vi "UHR-Fleezers Control (host) - 12.0(oscillate_test).vi"() -> ()   [LabVIEW 2014] (continued)
        n1707 = Concatenate Strings("User: ", "User", "\r", "Parameters saved.") -> (w2416:string)
        n1708 = call "Update messages.vi"("Message to add"=w2416, "Old message string"=w2421) -> ("New message string"=w2415:string)
        n1709 = local write "Messages"(w2415) -> ()
      }
      event "Load user params": Value Change {
        n1710 = event-data() -> ()  [unwired: 7 out]
        n1711 = local write "Load user params"(FALSE ("Read user\nparams")) -> ()
        n1712 = flat-sequence {
          tunnel: [w2453] -> w2441
          tunnel: [w2452] -> w2439
          tunnel: [w2451] -> w2437
          tunnel: [w2450] -> w2435
          tunnel: [w2449] -> w2433
          tunnel: [w2448] -> w2431
          tunnel: [w2447] -> w2429
          tunnel: [w2446] -> w2427
          tunnel: [w2445] -> w2425
          tunnel: [w2444] -> w2423
          tunnel: [w2463] -> w2442
          tunnel: w2441 -> [w2463]
          tunnel: [w2462] -> w2440
          tunnel: w2439 -> [w2462]
          tunnel: [w2461] -> w2438
          tunnel: w2437 -> [w2461]
          tunnel: [w2460] -> w2436
          tunnel: w2435 -> [w2460]
          tunnel: [w2459] -> w2434
          tunnel: w2433 -> [w2459]
          tunnel: [w2458] -> w2432
          tunnel: w2431 -> [w2458]
          tunnel: [w2457] -> w2430
          tunnel: w2429 -> [w2457]
          tunnel: [w2456] -> w2428
          tunnel: w2427 -> [w2456]
          tunnel: [w2455] -> w2426
          tunnel: w2425 -> [w2455]
          tunnel: [w2454] -> w2424
          tunnel: w2423 -> [w2454]
          tunnel: w2442 -> [w2480]
          tunnel: w2440 -> [w2479]
          tunnel: w2438 -> [w2478]
          tunnel: w2436 -> [w2477]
          tunnel: w2434 -> [w2476]
          tunnel: w2432 -> [w2475]
          tunnel: w2430 -> [w2474]
          tunnel: w2428 -> [w2473]
          tunnel: w2426 -> [w2472]
          tunnel: w2424 -> [w2471]
          frame #0 {
            # "Make exceptions.\nThese will not be\nloaded."
            n1713 = local read "Sample Channel\nFlow"() -> (w2448:bool)
            n1714 = local read "Green ON/Interlacing"() -> (w2449:bool)
            n1715 = local read "Trap 1 (ON/OFF)"() -> (w2453:bool)
            n1716 = local read "Trap 2 (ON/OFF)"() -> (w2452:bool)
            n1717 = local read "Trap Pos. FB ON"() -> (w2444:bool)
            n1718 = local read "Inject Pump 1"() -> (w2447:bool)
            n1719 = local read "Inject Pump 3"() -> (w2446:bool)
            n1720 = local read "Trap D (MHz)"() -> (w2445:dbl)
            n1721 = local read "Index"() -> (w2450:dbl)
            n1722 = local read "Fish"() -> (w2451:bool)
          }
          frame #1 {
            n1723 = local read "User"() -> (w2464:string)
            n1724 = call "retrieve control values.vi"("User"=w2464) -> ()  [unwired: 10 in, 1 out]
            n1725 = local read "Messages"() -> (w2470:string)
            n1726 = Concatenate Strings("User: ", w2464, "\r", "Parameters loaded.") -> (w2465:string)
            n1727 = call "Update messages.vi"("Message to add"=w2465, "Old message string"=w2470) -> ("New message string"=w2469:string)
            n1728 = local write "Messages"(w2469) -> ()
          }
          frame #2 {
            n1729 = local write "Sample Channel\nFlow"(w2475) -> ()
            n1730 = local write "Green ON/Interlacing"(w2476) -> ()
            n1731 = local write "Trap 1 (ON/OFF)"(w2480) -> ()
            n1732 = local write "Trap 2 (ON/OFF)"(w2479) -> ()
            n1733 = local write "Inject Pump 1"(w2474) -> ()
            n1734 = local write "Trap Pos. FB ON"(w2471) -> ()
            n1735 = local write "Inject Pump 3"(w2473) -> ()
            n1736 = local write "Trap D (MHz)"(w2472) -> ()
            n1737 = local write "Index"(w2477) -> ()
            n1738 = local write "Fish"(w2478) -> ()
          }
        }
      }
      event "Abort wiggle": Value Change {
        n1739 = event-data() -> ()  [unwired: 7 out]
        n1740 = flat-sequence {
          tunnel: w2484 -> [w2488]
          tunnel: w2483 -> [w2487]
          tunnel: [w2486] -> w2481
          tunnel: [w2490] -> w2482
          tunnel: w2481 -> [w2490]
          frame #0 {
            n1741 = xnode "Read/Write Control"("FPGA VI Reference In"=w2488, "error in"=w2487, "Abort wiggle 1"="Abort wiggle", "Abort wiggle 2"="Abort wiggle") -> ("error out"=w2486:errorcluster)  [unwired: 1 out]
          }
          frame #1 {
            n1742 = local write "Abort wiggle"(FALSE ("Abort wiggle")) -> ()
          }
        }
      }
    }
    "error out 2" <- w1261
    n1743 = node-c288() -> ()  [unwired: 2 out]
  }
  n1744 = node-c288() -> (w126:T26)  [unwired: 4 in]
  n1745 = local write "Target size"(cluster{"Width":dbl, "Height":dbl} {"Width"=40.0, "Height"=40.0} ("Target size")) -> ()
  n1746 = timed-loop "Run Scripts, including: stage motion" {
    tunnel: w130 -> [w2498]
    tunnel: w5 -> [w2499]
    tunnel: [w2499] -> w129
    tunnel: [w2498] -> w128
    timing: w126 -> [_]
    timing-out: [_] -> w125
    tunnel: w111 -> [w2497]
    tunnel: w112 -> [w2496]
    tunnel: w55 -> [w2493]
    tunnel: w54 -> [w2492]
    tunnel: w53 -> [w2494]
    tunnel: w52 -> [w2495]
    stop <- w2491 stop-if-true
    n1747 = node-c288() -> ()  [unwired: 1 in, 1 out]
    n1748 = event shown="[12] \"Got ADig bead\": Value Change" {
      selector: _ -> [_ _ _ _ _ _ _ _ _ _ _ _ _ _ _ _ _ _ _ _ _]
      dyn-events: _ -> [_ _ _ _ _ _ _ _ _ _ _ _ _ _ _ _ _ _ _ _ _]
      timeout: _ -> [_ _ _ _ _ _ _ _ _ _ _ _ _ _ _ _ _ _ _ _ _]
      tunnel: ["Set Position" "Move to Position" _ _ "Read Harvard" _ _ _ _ _ _ _ "Got ADig bead" "Force FB Script" "Rupture Script" _ "Got DNA bead" "Take Stepping Data" _ "Take Detection Laser\nImage" _] -> _
      tunnel: [_ _ _ _ _ _ _ _ _ _ _ _ _ _ _ _ _ _ _ _ w3172] -> w2491
      tunnel: w2498 -> [w2517 w2525 w2538 w2568 _ w2616 w2656 w2739 w2770 w2904 w2930 w2965 _ w2983 _ _ _ _ _ _ _]
      tunnel: w2499 -> [w2518 w2526 w2539 w2569 _ w2617 w2657 w2740 w2771 w2905 w2931 w2966 _ w2984 _ _ _ _ _ _ _]
      tunnel: w2497 -> [_ _ _ _ w2601 _ _ _ _ _ _ _ _ _ _ _ _ _ _ _ _]
      tunnel: w2496 -> [_ _ _ _ w2600 _ _ _ _ _ _ _ _ _ _ _ _ _ _ _ _]
      tunnel: w2495 -> [_ _ _ _ _ _ _ _ _ _ _ _ _ _ _ _ _ _ _ _ _]
      tunnel: w2494 -> [_ _ _ _ _ _ _ _ _ _ _ _ _ _ _ _ _ _ _ _ _]
      tunnel: w2493 -> [_ _ _ _ _ _ _ _ _ _ _ _ _ _ _ _ _ _ _ _ _]
      tunnel: w2492 -> [_ _ _ _ _ _ _ _ _ _ _ _ _ _ _ _ _ _ _ _ _]
      event "Set Position", "Set Position 2", "Set Position 3", "Set Position 4", "Set Position 5", "Set Position 1": Value Change {
        n1749 = event-data() -> ()  [unwired: 1 in, 5 out]
        n1750 = Build Array("Set Position 1", "Set Position 2", "Set Position 3", "Set Position 4", "Set Position 5") -> (w2516:bool[])
        n1751 = Boolean Array To Number(Boolean array=w2516) -> (number=w2515:u32)
        n1752 = Logarithm Base 2(1:w2515) -> (0:w2507:dbl)
        n1753 = call "Read Stage Position.vi"("error in"=w2517, "VISA resource name in"=w2518) -> ("Current Position"=w2522:cluster{dbl, dbl, dbl}, "error out"=w2521:errorcluster)  [unwired: 2 out]
        n1754 = Decrement(x="Position") -> (x-1=w2505:dbl)
        n1755 = Greater Or Equal?(x=w2507, y=0.0) -> (x >= y?=w2508:bool)
        n1756 = Cluster To Array(cluster=w2522) -> (array=w2519:dbl[])
        n1757 = local write "Stage Control Serial Error"(w2521) -> ()
        n1758 = Select(t=w2507, s=w2508, f=w2505) -> (s? t:f=w2504:dbl)
        n1759 = Increment(x=w2504) -> (x+1=w2503:dbl)
        n1760 = Build Array (concatenate)(w2503, w2519) -> (w2502:dbl[])
        n1761 = Replace Array Subset(array="Saved Stage Positions", new element=w2502, index (row)=w2504) -> (w2520:dbl[][])  [unwired: 1 in]
        n1762 = local write "Saved Stage Positions"(w2520) -> ()
      }
      event "Move to Position": Value Change {
        n1763 = event-data() -> ()  [unwired: 1 in, 5 out]
        n1764 = flat-sequence {
          tunnel: w2526 -> [w2530]
          tunnel: w2525 -> [w2529]
          frame #0 {
            n1765 = local read "Saved Stage Positions"() -> (w2532:dbl[][])
            n1766 = local read "Position"() -> (w2531:dbl)
            n1767 = local write "Stage Moving"(TRUE ("Stage Moving")) -> ()
            n1768 = call "move to saved stage position.vi"("error in"=w2529, "Stage VISA resource name in"=w2530, "Position"=w2531, "Saved Stage Positions"=w2532) -> ("error out"=w2528:errorcluster)  [unwired: 1 out]
            n1769 = local write "Stage Control Serial Error"(w2528) -> ()
          }
          frame #1 {
            n1770 = call <vilib>:"Beep.vi"() -> ()  [unwired: 3 in, 9 out]
            n1771 = local write "Stage Moving"(FALSE ("Stage Moving")) -> ()
          }
        }
      }
      event "Move Cap. 1 (DNA Bottom)": Value Change {
        n1772 = event-data() -> ()  [unwired: 1 in, 5 out]
        n1773 = local write "Move Cap. 1 (DNA Bottom)"(FALSE ("Move Cap. 1 (DNA Right)")) -> ()
        n1774 = flat-sequence {
          tunnel: w2538 -> [w2541]
          tunnel: w2539 -> [w2542]
          tunnel: [w2542] -> w2536
          tunnel: [w2541] -> w2535
          tunnel: w2536 -> [w2544]
          tunnel: w2535 -> [w2543]
          frame #0 {
            n1775 = property on="Sample Channel\nFlow" class="Bool (strict)"("Val(Sgnl)"="Cap 1 Samp Flow ON") -> ()  [unwired: 2 in, 2 out]
          }
          frame #1 {
            n1776 = local read "Saved Stage Positions"() -> (w2554:dbl[][])
            n1777 = local write "Stage Moving"(TRUE ("Stage Moving")) -> ()
            n1778 = Array Subset(array=w2554, index (row)=0 ("index"), length (row)=1 ("length"), index (col)=1 ("index"), length (col)=3 ("length")) -> (w2551:dbl[][])
            n1779 = Reshape Array(w2551, 3 ("dimension size")) -> (w2549:dbl[])
            n1780 = Array To Cluster(array=w2549) -> (cluster=w2548:cluster{"[0]":dbl, "[1]":dbl, "[2]":dbl})
            n1781 = call "Set Stage Position.vi"("Position"=w2548, "error in"=w2543, "VISA resource name in"=w2544) -> ("error out"=w2547:errorcluster)  [unwired: 2 out]
            n1782 = local write "Stage Control Serial Error"(w2547) -> ()
          }
          frame #2 {
            n1783 = local write "Stage Moving"(FALSE ("Stage Moving")) -> ()
            n1784 = case shown="True" "Cap 1 Flow ON" {
              frame False {
              }
              frame True {
                n1785 = property on="Inject Pump 1" class="Bool (strict)"("Val(Sgnl)"=TRUE ("Value (Signaling)")) -> ()  [unwired: 2 in, 2 out]
              }
            }
            n1786 = call <vilib>:"Beep.vi"() -> ()  [unwired: 3 in, 9 out]
          }
          frame #3 {
            n1787 = property on="Sample Channel\nFlow" class="Bool (strict)"("Val(Sgnl)"=FALSE ("Value (Signaling)")) -> ()  [unwired: 2 in, 2 out]
            n1788 = local read "Cap. 2 BD T1?\n(ADig T1, DNA T2)"() -> (w2561:bool)
            n1789 = case shown="True" w2561 {
              tunnel: "Cap 1 T ON" -> [w2563 w2564]
              frame False {
                n1790 = property on="Trap 1 (ON/OFF)" class="Bool (strict)"("Val(Sgnl)"=w2563) -> ()  [unwired: 2 in, 2 out]
              }
              frame True {
                n1791 = property on="Trap 2 (ON/OFF)" class="Bool (strict)"("Val(Sgnl)"=w2564) -> ()  [unwired: 2 in, 2 out]
              }
            }
            n1792 = property on="Got DNA bead" class="Bool (strict)"("Key Focus"=TRUE) -> ()  [unwired: 2 in, 2 out]
          }
        }
      }
      event "Move Cap. 2 (ADig Top)": Value Change {
        n1793 = event-data() -> ()  [unwired: 1 in, 5 out]
        n1794 = local write "Move Cap. 2 (ADig Top)"(FALSE ("Move Cap. 2 (ADig Left)")) -> ()
        n1795 = flat-sequence {
          tunnel: w2568 -> [w2571]
          tunnel: w2569 -> [w2572]
          tunnel: [w2572] -> w2566
          tunnel: [w2571] -> w2565
          tunnel: w2566 -> [w2574]
          tunnel: w2565 -> [w2573]
          frame #0 {
            n1796 = property on="Sample Channel\nFlow" class="Bool (strict)"("Val(Sgnl)"="Cap 2 Samp Flow ON") -> ()  [unwired: 2 in, 2 out]
          }
          frame #1 {
            n1797 = local read "Saved Stage Positions"() -> (w2584:dbl[][])
            n1798 = local write "Stage Moving"(TRUE ("Stage Moving")) -> ()
            n1799 = Array Subset(array=w2584, index (row)=1 ("index"), length (row)=1 ("length"), index (col)=1 ("index"), length (col)=3 ("length")) -> (w2581:dbl[][])
            n1800 = disable-structure shown="Disabled" {
              frame Disabled {
                w2586 = FALSE ("Value (Signaling)")
                n1801 = property on="Trap 1 (ON/OFF)" class="Bool (strict)"("Val(Sgnl)"=w2586) -> ()  [unwired: 2 in, 2 out]
                n1802 = property on="Trap 1 (ON/OFF)" class="Bool (strict)"("Val(Sgnl)"=w2586) -> ()  [unwired: 2 in, 2 out]
              }
              frame Enabled {
              }
            }
            n1803 = Reshape Array(w2581, 3 ("dimension size")) -> (w2579:dbl[])
            n1804 = Array To Cluster(array=w2579) -> (cluster=w2578:cluster{"[0]":dbl, "[1]":dbl, "[2]":dbl})
            n1805 = call "Set Stage Position.vi"("Position"=w2578, "error in"=w2573, "VISA resource name in"=w2574) -> ("error out"=w2577:errorcluster)  [unwired: 2 out]
            n1806 = local write "Stage Control Serial Error"(w2577) -> ()
          }
          frame #2 {
            n1807 = local write "Stage Moving"(FALSE ("Stage Moving")) -> ()
            n1808 = call <vilib>:"Beep.vi"() -> ()  [unwired: 3 in, 9 out]
            n1809 = case shown="True" "Cap 2 Flow ON" {
              frame False {
              }
              frame True {
                n1810 = property on="Inject Pump 3" class="Bool (strict)"("Val(Sgnl)"=TRUE ("Value (Signaling)")) -> ()  [unwired: 2 in, 2 out]
              }
            }
          }
          frame #3 {
            n1811 = Wait (ms)(milliseconds to wait=u32 500) -> ()  [unwired: 1 out]
          }
          frame #4 {
            n1812 = local read "Cal @ (MHz)"() -> (w2592:dbl)
            n1813 = property on="Sample Channel\nFlow" class="Bool (strict)"("Val(Sgnl)"=FALSE ("Value (Signaling)")) -> ()  [unwired: 2 in, 2 out]
            n1814 = case shown="False" "Cap. 2 BD T1?\n(ADig T1, DNA T2)" {
              tunnel: "Cap 2 T ON" -> [w2597 w2598]
              frame False {
                n1815 = property on="Trap 2 (ON/OFF)" class="Bool (strict)"("Val(Sgnl)"=w2597) -> ()  [unwired: 2 in, 2 out]
              }
              frame True {
                n1816 = property on="Trap 1 (ON/OFF)" class="Bool (strict)"("Val(Sgnl)"=w2598) -> ()  [unwired: 2 in, 2 out]
              }
            }
            n1817 = property on="Got ADig bead" class="Bool (strict)"("Key Focus"=TRUE) -> ()  [unwired: 2 in, 2 out]
            n1818 = local write "Target"("Target\nON?") -> ()
            n1819 = property on="Trap D (MHz)" class="DigNum (strict)"("Val(Sgnl)"=w2592) -> ()  [unwired: 2 in, 2 out]
          }
        }
      }
      event "Read Harvard": Value Change {
        n1820 = event-data() -> ()  [unwired: 1 in, 5 out]
        n1821 = Concatenate Strings("write buffer", "\r") -> (w2603:string)
        n1822 = VISA Write(VISA resource name=w2601, write buffer=w2603, error in (no error)=w2600) -> (VISA resource name out=w2612:refnum<visa-resource-name>, error out=w2611:errorcluster)  [unwired: 1 out]
        n1823 = stacked-sequence {
          tunnel: [w2615] -> w2610
          tunnel: w2612 -> [w2615]
          tunnel: w2611 -> [w2614]
          tunnel: [w2614] -> w2605
          frame #0 {
            n1824 = Wait (ms)(milliseconds to wait=50) -> ()  [unwired: 1 out]
          }
        }
        n1825 = property class="Instr"(reference=w2610, error in=w2605) -> (reference out=w2609:refnum<visa-resource-name>, error out=w2607:errorcluster, "Serial Settings:Number of Bytes at Serial Port"=w2608:u32)
        "Serial Settings:Number of Bytes at Serial Port" <- w2608
        n1826 = VISA Read(VISA resource name=w2609, byte count=w2608, error in (no error)=w2607) -> (read buffer=w2606:string)  [unwired: 3 out]
        "read buffer" <- w2606
        n1827 = Fract/Exp String To Number(string=w2606) -> ()  [unwired: 5 out]
      }
      event "+z", "-z": Value Change {
        n1828 = event-data() -> ()  [unwired: 1 in, 5 out]
        n1829 = flat-sequence {
          tunnel: w2616 -> [w2638]
          tunnel: w2617 -> [w2618]
          frame #0 {
            n1830 = call "Read Stage Position.vi"("error in"=w2638, "VISA resource name in"=w2618) -> ("Current Position"=w2623:cluster{dbl, dbl, dbl}, "error out"=w2636:errorcluster, "VISA resource name out"=w2637:refnum<visa-resource-name>)  [unwired: 1 out]
            n1831 = local read "Saved Stage Positions"() -> (w2647:dbl[][])
            n1832 = Divide(x="z nudge increment (um)", y=1000.0) -> (x/y=w2635:dbl)
            n1833 = Boolean To (0,1)(Boolean="+z") -> (0, 1=w2627:i16)
            n1834 = Boolean To (0,1)(Boolean="-z") -> (0, 1=w2628:i16)
            n1835 = Array Subset(array=w2647, index (row)=1 ("index"), length (row)=1 ("length"), index (col)=1 ("index"), length (col)=3 ("length")) -> (w2644:dbl[][])
            n1836 = Multiply(x=w2627, y=w2635) -> (x*y=w2631:dbl)
            n1837 = Multiply(x=w2628, y=w2635) -> (x*y=w2629:dbl)
            n1838 = Unbundle(w2623) -> (w2621:dbl, w2620:dbl, w2624:dbl)
            n1839 = Negate(x=w2629) -> (-x=w2630:dbl)
            n1840 = Reshape Array(w2644, 3 ("dimension size")) -> (w2642:dbl[])
            n1841 = Add(x=w2631, y=w2630) -> (x+y=w2632:dbl)
            n1842 = Array To Cluster(array=w2642) -> ()  [unwired: 1 out]
            n1843 = Add(x=w2632, y=w2624) -> (x+y=w2622:dbl)
            n1844 = Bundle(cluster=w2623, w2621, w2620, w2622) -> (w2619:cluster{dbl, dbl, dbl})
            n1845 = call "Set Stage Position.vi"("Position"=w2619, "error in"=w2636, "VISA resource name in"=w2637) -> ("error out"=w2641:errorcluster)  [unwired: 2 out]
            n1846 = local write "Stage Moving"(TRUE ("Stage Moving")) -> ()
            n1847 = local write "Stage Control Serial Error"(w2641) -> ()
          }
          frame #1 {
            n1848 = local write "Stage Moving"(FALSE ("Stage Moving")) -> ()
            n1849 = call <vilib>:"Beep.vi"() -> ()  [unwired: 3 in, 9 out]
          }
        }
      }
      event "Cal/Data Acq. Spot": Value Change {
        n1850 = event-data() -> ()  [unwired: 1 in, 5 out]
        n1851 = flat-sequence {
          tunnel: w2656 -> [w2660]
          tunnel: w2657 -> [w2661]
          tunnel: [w2661] -> w2653
          tunnel: [w2660] -> w2652
          tunnel: w2653 -> [w2666]
          tunnel: w2652 -> [w2665]
          tunnel: ["Cal @ (MHz)"] -> w2650
          tunnel: [w2670] -> w2654
          tunnel: w2650 -> [w2670]
          tunnel: w2654 -> [w2681]
          tunnel: ["W/ Offset 1"] -> w2651
          tunnel: w2654 -> [w2702]
          tunnel: w2651 -> [w2700]
          frame #0 {
            n1852 = property on="Sample Channel\nFlow" class="Bool (strict)"("Val(Sgnl)"="Daq spot flow on") -> ()  [unwired: 2 in, 2 out]
            n1853 = Wait (ms)(milliseconds to wait=u32 250) -> ()  [unwired: 1 out]
          }
          frame #1 {
            n1854 = local read "Saved Stage Positions"() -> (w2663:dbl[][])
            n1855 = property on="Trap D (MHz)" class="DigNum (strict)"("Val(Sgnl)"="Cal @ (MHz)") -> ()  [unwired: 2 in, 2 out]
            n1856 = local write "Stage Moving"(TRUE ("Stage Moving")) -> ()
            n1857 = call "move to saved stage position.vi"("error in"=w2665, "Stage VISA resource name in"=w2666, "Position"="Cal Stage Position", "Saved Stage Positions"=w2663) -> ("error out"=w2664:errorcluster)  [unwired: 1 out]
            n1858 = local write "Stage Control Serial Error"(w2664) -> ()
          }
          frame #2 {
            n1859 = local write "Stage Moving"(FALSE ("Stage Moving")) -> ()
            n1860 = property on="Sample Channel\nFlow" class="Bool (strict)"("Val(Sgnl)"="Flow ON\nduring cal?") -> ()  [unwired: 2 in, 2 out]
            n1861 = call <vilib>:"Beep.vi"() -> ()  [unwired: 3 in, 9 out]
          }
          frame #3 {
            n1862 = local read "Wait Before Save (s)"() -> (w2673:u32)
            n1863 = Multiply(x=w2673, y=u32 1000 ("milliseconds to wait")) -> (x*y=w2674:u32)
            n1864 = Wait (ms)(milliseconds to wait=w2674) -> ()  [unwired: 1 out]
          }
          frame #4 {
            n1865 = property on="Save Calibration" class="Bool (strict)"("Val(Sgnl)"=TRUE ("Value (Signaling)")) -> ()  [unwired: 2 in, 2 out]
          }
          frame #5 {
            n1866 = Wait (ms)(milliseconds to wait=u32 2000) -> ()  [unwired: 1 out]
          }
          frame #6 {
            # "Check to see if \nsaving done"
            n1867 = while {
              stop <- w2677 stop-if-true
              n1868 = local read "Saving..."() -> (w2678:bool)
              n1869 = Wait (ms)(milliseconds to wait=u32 100) -> ()  [unwired: 1 out]
              n1870 = Not(x=w2678) -> (.not. x?=w2677:bool)
            }
          }
          frame #7 {
            n1871 = case shown="True" "W/ Offset 1" {
              tunnel: w2681 -> [_ w2682]
              frame False {
              }
              frame True {
                n1872 = stacked-sequence {
                  tunnel: w2682 -> [_ _ _ _ _ _ _ w2699]
                  frame #0 {
                    n1873 = property on="Trap D (MHz)" class="DigNum (strict)"("Val(Sgnl)"="Offset 1 Start (MHz)") -> ()  [unwired: 2 in, 2 out]
                    n1874 = Replace Array Subset(array=u32[] [0] ("Index Values"), new element="Offset 1 Set", index=0) -> (w2683:u32[])
                    n1875 = property on="Saved AOD Raster Scan Parameter Sets" class="Arr (strict)"("Index Values"=w2683) -> ()  [unwired: 2 in, 2 out]
                  }
                  frame #1 {
                    n1876 = Wait (ms)(milliseconds to wait=u32 200) -> ()  [unwired: 1 out]
                  }
                  frame #2 {
                    n1877 = property on="Load parameters" class="Bool (strict)"("Val(Sgnl)"=TRUE ("Value (Signaling)")) -> ()  [unwired: 2 in, 2 out]
                  }
                  frame #3 {
                    n1878 = Wait (ms)(milliseconds to wait=u32 200) -> ()  [unwired: 1 out]
                  }
                  frame #4 {
                    n1879 = property on="Trap Raster Scan" class="Bool (strict)"("Val(Sgnl)"=TRUE ("Value (Signaling)")) -> ()  [unwired: 2 in, 2 out]
                  }
                  frame #5 {
                    n1880 = Wait (ms)(milliseconds to wait=u32 2000) -> ()  [unwired: 1 out]
                  }
                  frame #6 {
                    n1881 = while {
                      stop <- w2696 stop-if-true
                      n1882 = local read "Raster Scanning..."() -> (w2698:bool)
                      n1883 = local read "Saving..."() -> (w2694:bool)
                      n1884 = Wait (ms)(milliseconds to wait=u32 100) -> ()  [unwired: 1 out]
                      n1885 = Not(x=w2694) -> (.not. x?=w2693:bool)
                      n1886 = Not(x=w2698) -> (.not. x?=w2695:bool)
                      n1887 = And(x=w2695, y=w2693) -> (x .and. y?=w2696:bool)
                    }
                  }
                  frame #7 {
                    n1888 = property on="Trap D (MHz)" class="DigNum (strict)"("Val(Sgnl)"=w2699) -> ()  [unwired: 2 in, 2 out]
                  }
                }
              }
            }
          }
          frame #8 {
            n1889 = local read "Save ave N"() -> (w2701:dbl)
            n1890 = case shown="False" "W/ Offset 2" {
              tunnel: w2702 -> [_ w2709]
              tunnel: w2701 -> [_ w2708]
              tunnel: w2700 -> [w2704 _]
              frame False {
                n1891 = case shown="False" w2704 {
                  frame False {
                    n1892 = Multiply(x="Cal read wait (s)", y=u32 1000 ("milliseconds to wait")) -> (x*y=w2706:u32)
                    n1893 = Wait (ms)(milliseconds to wait=w2706) -> ()  [unwired: 1 out]
                  }
                  frame True {
                  }
                }
              }
              frame True {
                n1894 = stacked-sequence {
                  tunnel: w2709 -> [_ _ _ _ _ _ _ _ _ w2730 _ _]
                  tunnel: w2708 -> [_ _ _ _ _ _ _ _ _ w2728 _ _]
                  frame #0 {
                    n1895 = property on="Save ave N" class="DigNum (strict)"("Val(Sgnl)"=1.0 ("Value (Signaling)")) -> ()  [unwired: 2 in, 2 out]
                  }
                  frame #1 {
                    n1896 = Wait (ms)(milliseconds to wait=u32 500) -> ()  [unwired: 1 out]
                  }
                  frame #2 {
                    n1897 = property on="Trap D (MHz)" class="DigNum (strict)"("Val(Sgnl)"="Offset 2 Start (MHz)") -> ()  [unwired: 2 in, 2 out]
                    n1898 = Replace Array Subset(array=u32[] [0] ("Index Values"), new element="Offset 2 Set", index=0) -> (w2714:u32[])
                    n1899 = property on="Saved AOD Raster Scan Parameter Sets" class="Arr (strict)"("Index Values"=w2714) -> ()  [unwired: 2 in, 2 out]
                  }
                  frame #3 {
                    n1900 = Wait (ms)(milliseconds to wait=u32 500) -> ()  [unwired: 1 out]
                  }
                  frame #4 {
                    n1901 = property on="Load parameters" class="Bool (strict)"("Val(Sgnl)"=TRUE ("Value (Signaling)")) -> ()  [unwired: 2 in, 2 out]
                  }
                  frame #5 {
                    n1902 = Wait (ms)(milliseconds to wait=u32 500) -> ()  [unwired: 1 out]
                  }
                  frame #6 {
                    n1903 = property on="Trap Raster Scan" class="Bool (strict)"("Val(Sgnl)"=TRUE ("Value (Signaling)")) -> ()  [unwired: 2 in, 2 out]
                  }
                  frame #7 {
                    n1904 = Wait (ms)(milliseconds to wait=u32 2000) -> ()  [unwired: 1 out]
                  }
                  frame #8 {
                    n1905 = while {
                      stop <- w2723 stop-if-true
                      n1906 = local read "Raster Scanning..."() -> (w2726:bool)
                      n1907 = local read "Saving..."() -> (w2724:bool)
                      n1908 = Wait (ms)(milliseconds to wait=u32 100) -> ()  [unwired: 1 out]
                      n1909 = Not(x=w2724) -> (.not. x?=w2722:bool)
                      n1910 = Not(x=w2726) -> (.not. x?=w2725:bool)
                      n1911 = And(x=w2725, y=w2722) -> (x .and. y?=w2723:bool)
                    }
                  }
                  frame #9 {
                    n1912 = property on="Trap D (MHz)" class="DigNum (strict)"("Val(Sgnl)"=w2730) -> ()  [unwired: 2 in, 2 out]
                    n1913 = property on="Saved AOD Raster Scan Parameter Sets" class="Arr (strict)"("Index Values"=u32[] [0]) -> ()  [unwired: 2 in, 2 out]
                    n1914 = property on="Save ave N" class="DigNum (strict)"("Val(Sgnl)"=w2728) -> ()  [unwired: 2 in, 2 out]
                  }
                  frame #10 {
                    n1915 = Wait (ms)(milliseconds to wait=u32 500) -> ()  [unwired: 1 out]
                  }
                  frame #11 {
                    n1916 = property on="Load parameters" class="Bool (strict)"("Val(Sgnl)"=TRUE ("Value (Signaling)")) -> ()  [unwired: 2 in, 2 out]
                  }
                }
              }
            }
          }
          frame #9 {
            n1917 = property on="Read Cal" class="Bool (strict)"("Val(Sgnl)"=TRUE ("Value (Signaling)")) -> ()  [unwired: 2 in, 2 out]
          }
          frame #10 {
            n1918 = Wait (ms)(milliseconds to wait=u32 1000) -> ()  [unwired: 1 out]
          }
          frame #11 {
            n1919 = property on="Fish" class="Bool (strict)"("Val(Sgnl)"=TRUE ("Value (Signaling)")) -> ()  [unwired: 2 in, 2 out]
          }
        }
        n1920 = local write "Cal/Data Acq. Spot"(FALSE ("Cal/Data Acq. Spot")) -> ()
      }
      event "Dump Beads": Value Change {
        n1921 = event-data() -> ()  [unwired: 1 in, 5 out]
        n1922 = flat-sequence {
          tunnel: ["Dump spot flow on?"] -> w2736
          tunnel: [w2748] -> w2737
          tunnel: w2736 -> [w2748]
          tunnel: w2740 -> [w2753]
          tunnel: w2739 -> [w2752]
          tunnel: [w2750] -> w2738
          tunnel: w2737 -> [w2750]
          tunnel: w2738 -> [w2764]
          frame #0 {
            w2741 = FALSE ("Value (Signaling)")
            n1923 = local read "Saving..."() -> (w2743:bool)
            n1924 = local write "Dump Beads"(FALSE ("Dump Beads")) -> ()
            n1925 = property on="Inject Pump 3" class="Bool (strict)"("Val(Sgnl)"=w2741) -> ()  [unwired: 2 in, 2 out]
            n1926 = property on="Inject Pump 1" class="Bool (strict)"("Val(Sgnl)"=w2741) -> ()  [unwired: 2 in, 2 out]
            n1927 = local write "Stop Saving"(w2743) -> ()
            n1928 = local write "Fish"(w2741) -> ()
          }
          frame #1 {
            w2744 = TRUE
            w2745 = FALSE ("Fl. Triggered...")
            n1929 = case shown="True" "Dump spot flow on?" {
              frame False {
              }
              frame True {
                n1930 = property on="Sample Channel\nFlow" class="Bool (strict)"("Val(Sgnl)"=TRUE ("Stage Moving")) -> ()  [unwired: 2 in, 2 out]
              }
            }
            n1931 = local write "Fl. Triggered..."(w2745) -> ()
            n1932 = local write "Tether"(w2745) -> ()
            n1933 = local write "Multiple tether"(w2745) -> ()
            n1934 = local write "Good tether"(w2745) -> ()
            n1935 = property on="Green ON/Interlacing" class="Bool (strict)"("Val(Sgnl)"=w2745) -> ()  [unwired: 2 in, 2 out]
            n1936 = property on="Trap Pos. FB ON" class="Bool (strict)"("Val(Sgnl)"=w2745) -> ()  [unwired: 2 in, 2 out]
            n1937 = property on="Trap Trig. Fl." class="Bool (strict)"("Val(Sgnl)"=w2745) -> ()  [unwired: 2 in, 2 out]
            n1938 = local write "Bad fit"(w2745) -> ()
            n1939 = local write "Hysteresis"(w2745) -> ()
            n1940 = property on="Fl. Triggered..." class="Bool (strict)"("Val(Sgnl)"=w2745) -> ()  [unwired: 2 in, 2 out]
            n1941 = local write "Restart DMA? (AOD)"(w2744) -> ()
            n1942 = local write "Save scans"(w2744) -> ()
            n1943 = property on="Dip for Protein" class="Bool (strict)"("Val(Sgnl)"=w2745) -> ()  [unwired: 2 in, 2 out]
            n1944 = property on="Pause dwell" class="Bool (strict)"("Val(Sgnl)"=w2745) -> ()  [unwired: 2 in, 2 out]
          }
          frame #2 {
            n1945 = property on="Trap Pos. FB Offset Factor" class="DigNum (strict)"("Val(Sgnl)"=i64 0 ("Value (Signaling)")) -> ()  [unwired: 2 in, 2 out]
          }
          frame #3 {
            n1946 = local read "Saved Stage Positions"() -> (w2754:dbl[][])
            n1947 = Array Subset(array=w2754, index (row)=3 ("index"), length (row)=1 ("length"), index (col)=1 ("index"), length (col)=3 ("length")) -> (w2759:dbl[][])
            n1948 = local write "Stage Moving"(TRUE ("Stage Moving")) -> ()
            n1949 = Reshape Array(w2759, 3 ("dimension size")) -> (w2757:dbl[])
            n1950 = Array To Cluster(array=w2757) -> (cluster=w2756:cluster{"[0]":dbl, "[1]":dbl, "[2]":dbl})
            n1951 = call "Set Stage Position.vi"("Position"=w2756, "error in"=w2752, "VISA resource name in"=w2753) -> ()  [unwired: 3 out]
          }
          frame #4 {
            w2765 = FALSE ("Value (Signaling)")
            n1952 = case shown="True" w2764 {
              frame False {
              }
              frame True {
                n1953 = property on="Sample Channel\nFlow" class="Bool (strict)"("Val(Sgnl)"=FALSE ("Stage Moving")) -> ()  [unwired: 2 in, 2 out]
              }
            }
            n1954 = property on="Trap 1 (ON/OFF)" class="Bool (strict)"("Val(Sgnl)"=w2765) -> ()  [unwired: 2 in, 2 out]
            n1955 = property on="Trap 2 (ON/OFF)" class="Bool (strict)"("Val(Sgnl)"=w2765) -> ()  [unwired: 2 in, 2 out]
            n1956 = call <vilib>:"Beep.vi"() -> ()  [unwired: 3 in, 9 out]
            n1957 = local write "Fish"(FALSE ("Fish for Tether")) -> ()
          }
          frame #5 {
            n1958 = property on="Move Cap. 2 (ADig Top)" class="Bool (strict)"("Val(Sgnl)"=TRUE ("Value (Signaling)")) -> ()  [unwired: 2 in, 2 out]
            n1959 = property on="Tab Control" class="TabCtl (strict)"("Val(Sgnl)"=T34."Status" ("Value (Signaling)")) -> ()  [unwired: 2 in, 2 out]
          }
        }
      }
      event "Dip for Protein": Value Change {
        n1960 = event-data() -> ()  [unwired: 1 in, 5 out]
        n1961 = case shown="True" "Dip for Protein" {
          tunnel: w2771 -> [_ w2773]
          tunnel: w2770 -> [_ w2772]
          frame False {
          }
          frame True {
            n1962 = while {
              tunnel: w2773 -> [w2784]
              tunnel: w2772 -> [w2783]
              i -> [w2779]
              stop <- w2774 stop-if-true
              n1963 = Increment(x=w2779) -> (x+1=→"Dip #":i32)
              n1964 = flat-sequence {
                tunnel: w2783 -> [w2795]
                tunnel: w2784 -> [w2796]
                tunnel: [w2796] -> w2788
                tunnel: [w2795] -> w2787
                tunnel: [w2789] -> w2775
                tunnel: [w2801] -> w2782
                tunnel: [w2802] -> w2781
                tunnel: w2788 -> [w2803]
                tunnel: w2787 -> [w2804]
                tunnel: [w2799] -> w2776
                tunnel: w2775 -> [w2799]
                tunnel: [w2812] -> w2786
                tunnel: w2782 -> [w2812]
                tunnel: [w2811] -> w2785
                tunnel: w2781 -> [w2811]
                tunnel: [w2808] -> w2780
                tunnel: [w2807] -> w2777
                tunnel: w2776 -> [w2807]
                tunnel: w2785 -> [w2832]
                tunnel: w2786 -> [w2833]
                tunnel: w2780 -> [w2834]
                tunnel: w2777 -> [w2831]
                tunnel: [w2893] -> w2774
                frame #0 {
                  n1965 = local read "Trap Pos. FB ON"() -> (w2789:bool)
                  n1966 = Compound Arithmetic op=AND("Flow ON\nduring dip?", "FB OFF when \nflow ON", w2789) -> (w2790:bool)
                  n1967 = case shown="True" "Move trap \nbefore dip move?" {
                    frame False {
                    }
                    frame True {
                      n1968 = property on="Trap D (MHz)" class="DigNum (strict)"("Val(Sgnl)"="Dipping D (MHz)") -> ()  [unwired: 2 in, 2 out]
                    }
                  }
                  n1969 = property on="Green ON/Interlacing" class="Bool (strict)"("Val(Sgnl)"="Green ON\nbefore dip?") -> ()  [unwired: 2 in, 2 out]
                  n1970 = property on="Sample Channel\nFlow" class="Bool (strict)"("Val(Sgnl)"="Flow ON\nduring dip?") -> ()  [unwired: 2 in, 2 out]
                  n1971 = case shown="True" w2790 {
                    frame False {
                    }
                    frame True {
                      n1972 = property on="Trap Pos. FB ON" class="Bool (strict)"("Val(Sgnl)"=FALSE ("Value (Signaling)")) -> ()  [unwired: 2 in, 2 out]
                    }
                  }
                }
                frame #1 {
                  n1973 = local read "Saved Stage Positions"() -> (w2806:dbl[][])
                  n1974 = local write "Cancel dwell"(FALSE ("Cancel dwell")) -> ()
                  n1975 = call "move to saved stage position.vi"("error in"=w2804, "Stage VISA resource name in"=w2803, "Position"="Dip Stage \nPosition", "Saved Stage Positions"=w2806) -> ("VISA resource name out"=w2801:refnum<visa-resource-name>, "error out"=w2802:errorcluster)
                }
                frame #2 {
                  n1976 = node-c288() -> (w2810:T26)  [unwired: 4 in]
                  n1977 = timed-loop {
                    timing: w2810 -> [_]
                    timing-out: [_] -> w2809
                    tunnel: [w2816] -> w2808
                    i -> [w2813]
                    stop <- w2817 stop-if-true
                    n1978 = node-c288() -> ()  [unwired: 1 in, 1 out]
                    n1979 = Greater Or Equal?(x=w2813, y="Dip Duration (s)") -> (x >= y?=w2825:bool)
                    n1980 = local read "Dip for Protein"() -> (w2818:bool)
                    n1981 = local read "Dump Beads"() -> (w2815:bool)
                    n1982 = local read "Cancel dwell"() -> (w2824:bool)
                    n1983 = local read "Pause dwell"() -> (w2821:bool)
                    n1984 = Not(x=w2818) -> (.not. x?=w2823:bool)
                    n1985 = Compound Arithmetic op=OR(w2824, w2825, w2823) -> (w2822:bool)
                    n1986 = Select(t=FALSE, s=w2821, f=w2822) -> (s? t:f=w2819:bool)
                    n1987 = Not(x=w2815) -> (.not. x?=w2814:bool)
                    n1988 = node-c288() -> ()  [unwired: 1 in, 1 out]
                    n1989 = And(x=w2818, y=w2814) -> (x .and. y?=w2816:bool)
                    n1990 = Or(x=w2819, y=w2815) -> (x .or. y?=w2817:bool)
                    "Dip Time (s)" <- w2813
                  }
                  n1991 = node-c288(w2809) -> ()  [unwired: 1 out]
                }
                frame #3 {
                  n1992 = case shown="True" w2834 {
                    tunnel: w2833 -> [_ w2839]
                    tunnel: w2832 -> [_ w2838]
                    tunnel: w2831 -> [_ w2835]
                    frame False {
                    }
                    frame True {
                      n1993 = flat-sequence {
                        tunnel: w2838 -> [w2843]
                        tunnel: w2839 -> [w2844]
                        tunnel: [w2844] -> w2837
                        tunnel: [w2843] -> w2836
                        tunnel: w2835 -> [w2840]
                        tunnel: w2837 -> [w2854]
                        tunnel: w2836 -> [w2853]
                        tunnel: w2835 -> [w2862]
                        frame #0 {
                          n1994 = local read "Sample Channel\nFlow"() -> (w2842:bool)
                          n1995 = case shown="True" w2842 {
                            tunnel: "Flow ON \nduring return\nfrom dip?" -> [w2845 w2848]
                            tunnel: w2840 -> [_ w2847]
                            frame False {
                              n1996 = case shown="True" w2845 {
                                frame False {
                                }
                                frame True {
                                n1997 = property on="Sample Channel\nFlow" class="Bool (strict)"("Val(Sgnl)"=TRUE ("Value (Signaling)")) -> ()  [unwired: 2 in, 2 out]
                                }
                              }
                            }
                            frame True {
                              n1998 = case shown="False" w2848 {
                                tunnel: w2847 -> [w2849 _]
                                frame False {
                                n1999 = property on="Trap Pos. FB ON" class="Bool (strict)"("Val(Sgnl)"=w2849) -> ()  [unwired: 2 in, 2 out]
                                n2000 = property on="Sample Channel\nFlow" class="Bool (strict)"("Val(Sgnl)"=FALSE ("Value (Signaling)")) -> ()  [unwired: 2 in, 2 out]
                                }
                                frame True {
                                }
                              }
                            }
                          }
                        }
                        frame #1 {
                          # "For turning on green laser before stage reaches lower spot"
                          n2001 = case shown="True" "Green ON\nafter start\nreturn?" {
                            frame False {
                            }
                            frame True {
                              n2002 = flat-sequence {
                                frame #0 {
                                n2003 = Multiply(x="Green delay after \nstart return (s)", y=1000.0) -> (x*y=w2859:dbl)
                                n2004 = Wait (ms)(milliseconds to wait=w2859) -> ()  [unwired: 1 out]
                                }
                                frame #1 {
                                n2005 = property on="Green ON/Interlacing" class="Bool (strict)"("Val(Sgnl)"=TRUE ("Value (Signaling)")) -> ()  [unwired: 2 in, 2 out]
                                }
                              }
                            }
                          }
                          n2006 = local read "Saved Stage Positions"() -> (w2857:dbl[][])
                          n2007 = local write "Cancel dwell"(FALSE ("Cancel dwell")) -> ()
                          n2008 = call "move to saved stage position.vi"("error in"=w2853, "Stage VISA resource name in"=w2854, "Position"="Return Stage \nPosition", "Saved Stage Positions"=w2857) -> ("error out"=w2855:errorcluster)  [unwired: 1 out]
                          n2009 = local write "Stage Control Serial Error"(w2855) -> ()
                        }
                        frame #2 {
                          n2010 = property on="Trap Pos. FB ON" class="Bool (strict)"("Val(Sgnl)"=w2862) -> ()  [unwired: 2 in, 2 out]
                          n2011 = case shown="True" "Green ON \nafter return?" {
                            frame False {
                            }
                            frame True {
                              n2012 = property on="Green ON/Interlacing" class="Bool (strict)"("Val(Sgnl)"=TRUE ("Value (Signaling)")) -> ()  [unwired: 2 in, 2 out]
                            }
                          }
                          n2013 = case shown="True" "Move trap after return?" {
                            frame False {
                            }
                            frame True {
                              n2014 = property on="Trap D (MHz)" class="DigNum (strict)"("Val(Sgnl)"="Dip Trap D 2 (MHz)") -> ()  [unwired: 2 in, 2 out]
                            }
                          }
                          n2015 = case shown="True" "Save data after return?" {
                            frame False {
                            }
                            frame True {
                              n2016 = property on="Start Saving" class="Bool (strict)"("Val(Sgnl)"=TRUE ("Value (Signaling)")) -> ()  [unwired: 2 in, 2 out]
                            }
                          }
                          n2017 = property on="Sample Channel\nFlow" class="Bool (strict)"("Val(Sgnl)"="Flow ON\nduring daq?") -> ()  [unwired: 2 in, 2 out]
                        }
                        frame #3 {
                          n2018 = node-c288() -> (w2871:T26)  [unwired: 4 in]
                          n2019 = timed-loop {
                            timing: w2871 -> [_]
                            timing-out: [_] -> w2870
                            i -> [w2872]
                            stop <- w2874 stop-if-true
                            n2020 = node-c288() -> ()  [unwired: 1 in, 1 out]
                            n2021 = local read "Dump Beads"() -> (w2873:bool)
                            n2022 = Greater Or Equal?(x=w2872, y="Dwell Duration (s)") -> (x >= y?=w2879:bool)
                            n2023 = local read "Dip for Protein"() -> (w2876:bool)
                            n2024 = Not(x=w2876) -> (.not. x?=w2875:bool)
                            n2025 = Compound Arithmetic op=OR(w2879, "Cancel dwell", w2875) -> (w2878:bool)
                            n2026 = node-c288() -> ()  [unwired: 1 in, 1 out]
                            n2027 = Select(t=FALSE, s="Pause dwell", f=w2878) -> (s? t:f=w2881:bool)
                            n2028 = Or(x=w2881, y=w2873) -> (x .or. y?=w2874:bool)
                            "Dwell Time (s)" <- w2872
                          }
                          n2029 = node-c288(w2870) -> ()  [unwired: 1 out]
                        }
                      }
                    }
                  }
                }
                frame #4 {
                  n2030 = local read "Dip for Protein"() -> (w2890:bool)
                  n2031 = local read "Tether"() -> (w2889:bool)
                  n2032 = local read "Dump Beads"() -> (w2891:bool)
                  n2033 = local write "Cancel dwell"(FALSE ("Cancel dwell")) -> ()
                  n2034 = Not(x=w2889) -> (.not. x?=w2888:bool)
                  n2035 = Not(x=w2890) -> (.not. x?=w2894:bool)
                  n2036 = Not(x="Cont. Repeat Dipping?") -> (.not. x?=w2896:bool)
                  n2037 = Compound Arithmetic op=OR(w2888, w2894, w2896, w2891) -> (w2893:bool)
                }
              }
            }
          }
        }
      }
      event "Profile": Value Change {
        n2038 = event-data() -> ()  [unwired: 1 in, 5 out]
        n2039 = flat-sequence {
          tunnel: w2905 -> [w2908]
          tunnel: w2904 -> [w2916]
          tunnel: [w2910] -> w2903
          tunnel: [w2909] -> w2902
          tunnel: [w2907] -> w2900
          tunnel: [w2906] -> w2897
          tunnel: w2903 -> [w2923]
          tunnel: w2902 -> [w2922]
          tunnel: [w2920] -> w2901
          tunnel: w2900 -> [w2921]
          tunnel: [w2919] -> w2899
          tunnel: [w2918] -> w2898
          tunnel: w2897 -> [w2918]
          tunnel: w2901 -> [w2927]
          tunnel: w2899 -> [w2926]
          tunnel: w2898 -> [w2925]
          frame #0 {
            n2040 = call "Read Stage Position.vi"("error in"=w2916, "VISA resource name in"=w2908) -> ("Current Position"=w2906:cluster{dbl, dbl, dbl}, "error out"=w2909:errorcluster, "VISA resource name out"=w2907:refnum<visa-resource-name>)  [unwired: 1 out]
            "Current Position" <- w2906
            n2041 = local write "Stage Control Serial Error"(w2909) -> ()
            n2042 = Unbundle(w2906) -> (w2913:dbl, w2915:dbl, w2911:dbl)
            n2043 = Add(x=w2915, y="Y change (mm)") -> (x+y=w2912:dbl)
            n2044 = Bundle(w2913, w2912, w2911) -> (w2910:cluster{dbl, dbl, dbl})  [unwired: 1 in]
          }
          frame #1 {
            # "move to new position and start saving"
            n2045 = local write "Stage Moving"(TRUE ("Stage Moving")) -> ()
            n2046 = local write "Start Saving"(TRUE ("Start Saving")) -> ()
            n2047 = call "Set Stage Position.vi"("Position"=w2923, "error in"=w2922, "VISA resource name in"=w2921) -> ("error out"=w2919:errorcluster, "VISA resource name out"=w2920:refnum<visa-resource-name>)  [unwired: 1 out]
          }
          frame #2 {
            # "go back to start"
            n2048 = call "Set Stage Position.vi"("Position"=w2925, "error in"=w2926, "VISA resource name in"=w2927) -> ()  [unwired: 3 out]
          }
          frame #3 {
            # "stop saving"
            n2049 = local write "Stop Saving"(TRUE ("Stop Saving")) -> ()
            n2050 = local write "Stage Moving"(FALSE ("Stage Moving")) -> ()
          }
        }
      }
      event "Move to Position 1", "Move to Position 2", "Move to Position 3", "Move to Position 4", "Move to Position 5", "Lower Ch. Cap.": Value Change {
        n2051 = event-data() -> ()  [unwired: 1 in, 5 out]
        n2052 = Or(x="Move to Position 5", y="Lower Ch. Cap.") -> (x .or. y?=w2933:bool)
        n2053 = Build Array("Move to Position 1", "Move to Position 2", "Move to Position 3", "Move to Position 4", w2933) -> (w2936:bool[])
        n2054 = Boolean Array To Number(Boolean array=w2936) -> (number=w2935:u32)
        n2055 = Logarithm Base 2(1:w2935) -> (0:w2934:dbl)
        n2056 = flat-sequence {
          tunnel: w2934 -> [w2945]
          tunnel: w2931 -> [w2943]
          tunnel: w2930 -> [w2942]
          frame #0 {
            n2057 = local read "Saved Stage Positions"() -> (w2953:dbl[][])
            n2058 = Array Subset(array=w2953, index (row)=w2945, length (row)=1 ("length"), index (col)=1 ("index"), length (col)=3 ("length")) -> (w2950:dbl[][])
            n2059 = Reshape Array(w2950, 3 ("dimension size")) -> (w2948:dbl[])
            n2060 = Array To Cluster(array=w2948) -> (cluster=w2947:cluster{"[0]":dbl, "[1]":dbl, "[2]":dbl})
            n2061 = call "Set Stage Position.vi"("Position"=w2947, "error in"=w2942, "VISA resource name in"=w2943) -> ("error out"=w2946:errorcluster)  [unwired: 2 out]
            n2062 = local write "Stage Moving"(TRUE ("Stage Moving")) -> ()
            n2063 = local write "Stage Control Serial Error"(w2946) -> ()
          }
          frame #1 {
            n2064 = local write "Stage Moving"(FALSE ("Stage Moving")) -> ()
            n2065 = call <vilib>:"Beep.vi"() -> ()  [unwired: 3 in, 9 out]
          }
        }
      }
      event "Set Current\nPos to 0,0,0": Value Change {
        # "DH is \"Define Home\""
        n2066 = event-data() -> ()  [unwired: 1 in, 6 out]
        n2067 = local write "Set Current\nPos to 0,0,0"(FALSE ("Set Current\nPos to 0,0,0")) -> ()
        n2068 = Concatenate Strings("1DH" ("string"), ";" ("string"), "2DH" ("string"), ";" ("string"), "3DH" ("string"), "\r") -> (w2961:string)
        n2069 = call-poly "VISA Configure Serial Port"("VISA resource name"=w2966, "baud rate (9600)"=u32 19200, "error in (no error)"=w2965) -> ("VISA resource name out"=w2963:refnum<visa-resource-name>, "error out"=w2962:errorcluster)  [unwired: 11 in]
        n2070 = VISA Write(VISA resource name=w2963, write buffer=w2961, error in (no error)=w2962) -> (error out=w2956:errorcluster)  [unwired: 2 out]
        n2071 = local write "Stage Control Serial Error"(w2956) -> ()
      }
      event "Got ADig bead": Value Change {
        n2072 = event-data() -> ()  [unwired: 1 in, 5 out]
        n2073 = flat-sequence {
          frame #0 {
            n2074 = local read "Cap 1 Samp Flow ON"() -> (w2972:bool)
            n2075 = case shown="True" w2972 {
              frame False {
              }
              frame True {
                n2076 = property on="Sample Channel\nFlow" class="Bool (strict)"("Val(Sgnl)"=TRUE ("Value (Signaling)")) -> ()  [unwired: 2 in, 2 out]
              }
            }
            n2077 = local write "Got ADig bead"(FALSE) -> ()
          }
          frame #1 {
            n2078 = property on="Inject Pump 3" class="Bool (strict)"("Val(Sgnl)"=FALSE ("Value (Signaling)")) -> ()  [unwired: 2 in, 2 out]
            n2079 = local write "Target"(FALSE ("Target")) -> ()
          }
          frame #2 {
            n2080 = property on="Move Cap. 1 (DNA Bottom)" class="Bool (strict)"("Val(Sgnl)"=TRUE ("Value (Signaling)")) -> ()  [unwired: 2 in, 2 out]
          }
        }
      }
      event "Force FB Script": Value Change {
        n2081 = event-data() -> ()  [unwired: 1 in, 5 out]
        n2082 = local write "Force FB Script"(FALSE ("Force FB Data\nScript")) -> ()
        n2083 = flat-sequence {
          tunnel: w2983 -> [w2987]
          tunnel: w2984 -> [w2988]
          tunnel: [w2988] -> w2979
          tunnel: [w2987] -> w2978
          tunnel: w2979 -> [w2991]
          tunnel: w2978 -> [w2990]
          tunnel: ["Trap Trig Fl."] -> w2980
          tunnel: [w3033] -> w2981
          tunnel: w2980 -> [w3033]
          tunnel: [w3037] -> w2982
          tunnel: w2981 -> [w3037]
          tunnel: w2982 -> [w3039]
          frame #0 {
            n2084 = property on="Trap D (MHz)" class="DigNum (strict)"("Val(Sgnl)"="Trap D Before Moving") -> ()  [unwired: 2 in, 2 out]
          }
          frame #1 {
            n2085 = local read "Saved Stage Positions"() -> (w2993:dbl[][])
            n2086 = local write "FB Trap Pos Offset"(0.0 ("FB Trap Pos Offset")) -> ()
            n2087 = property on="Trap Pos. FB Offset Factor" class="DigNum (strict)"("Val(Sgnl)"=i64 0 ("Value (Signaling)")) -> ()  [unwired: 2 in, 2 out]
            n2088 = local write "Stage Moving"(TRUE ("Stage Moving")) -> ()
            n2089 = call "move to saved stage position.vi"("error in"=w2990, "Stage VISA resource name in"=w2991, "Position"="Stage Position To Establish FB", "Saved Stage Positions"=w2993) -> ("error out"=w2989:errorcluster)  [unwired: 1 out]
            n2090 = local write "Stage Control Serial Error"(w2989) -> ()
          }
          frame #2 {
            n2091 = call <vilib>:"Beep.vi"("duration (msec)"=u32 100, "frequency (Hz)"=u32 20) -> ()  [unwired: 1 in, 9 out]
            n2092 = local write "Stage Moving"(FALSE ("Stage Moving")) -> ()
            n2093 = property on="Tab Control 2" class="TabCtl (strict)"("Val(Sgnl)"=T6."Feedback on Trap Position" ("Value (Signaling)")) -> ()  [unwired: 2 in, 2 out]
            n2094 = stacked-sequence {
              frame #0 {
                n2095 = Multiply(x="Wait (s)", y=u32 1000 ("milliseconds to wait")) -> (x*y=w3002:u32)
                n2096 = property on="Trap D (MHz)" class="DigNum (strict)"("Val(Sgnl)"="Starting Trap D (MHz)") -> ()  [unwired: 2 in, 2 out]
                n2097 = Wait (ms)(milliseconds to wait=w3002) -> ()  [unwired: 1 out]
              }
              frame #1 {
                n2098 = property on="Set Reading to\nSetpoint" class="Bool (strict)"("Val(Sgnl)"=TRUE ("Value (Signaling)")) -> ()  [unwired: 2 in, 2 out]
              }
            }
            n2099 = property on="Tab Control" class="TabCtl (strict)"("Val(Sgnl)"=T34."Trap Control (RF)" ("Value (Signaling)")) -> ()  [unwired: 2 in, 2 out]
          }
          frame #3 {
            n2100 = Wait (ms)(milliseconds to wait=u32 500) -> ()  [unwired: 1 out]
          }
          frame #4 {
            n2101 = property on="Trap Pos. FB ON" class="Bool (strict)"("Val(Sgnl)"=TRUE ("Value (Signaling)")) -> ()  [unwired: 2 in, 2 out]